vi "45-1523-1 State Diagram.vi"() -> ()   [LabVIEW 2015] (continued)
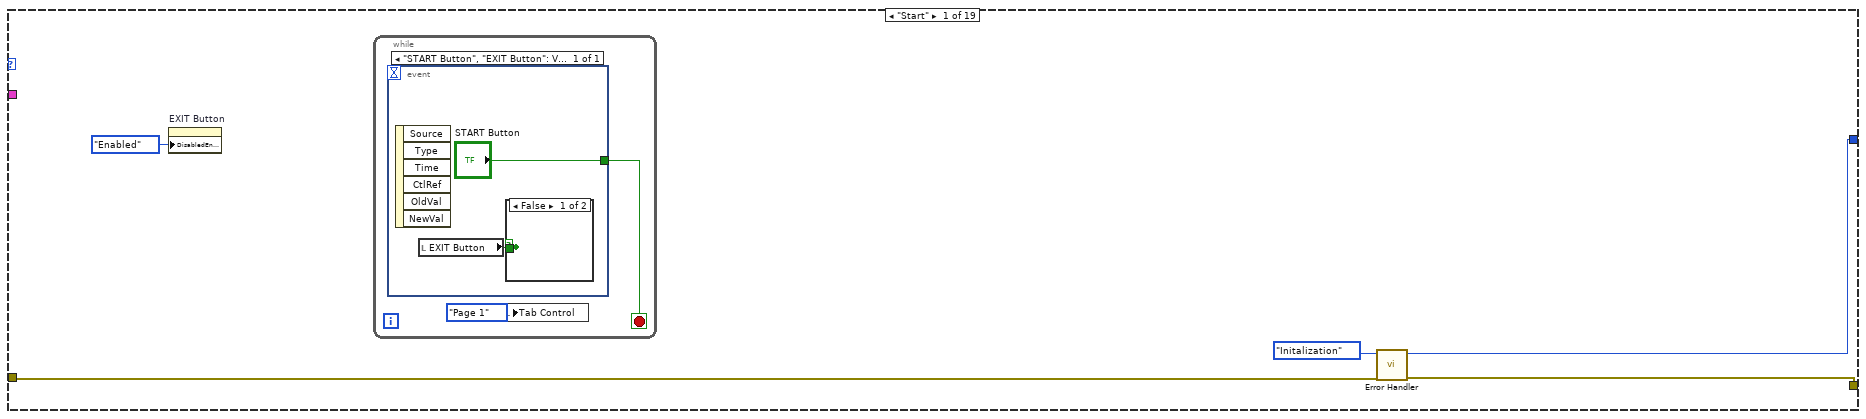
[diagram p2: hidden frame]
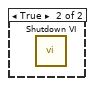
[diagram p3: hidden frame]
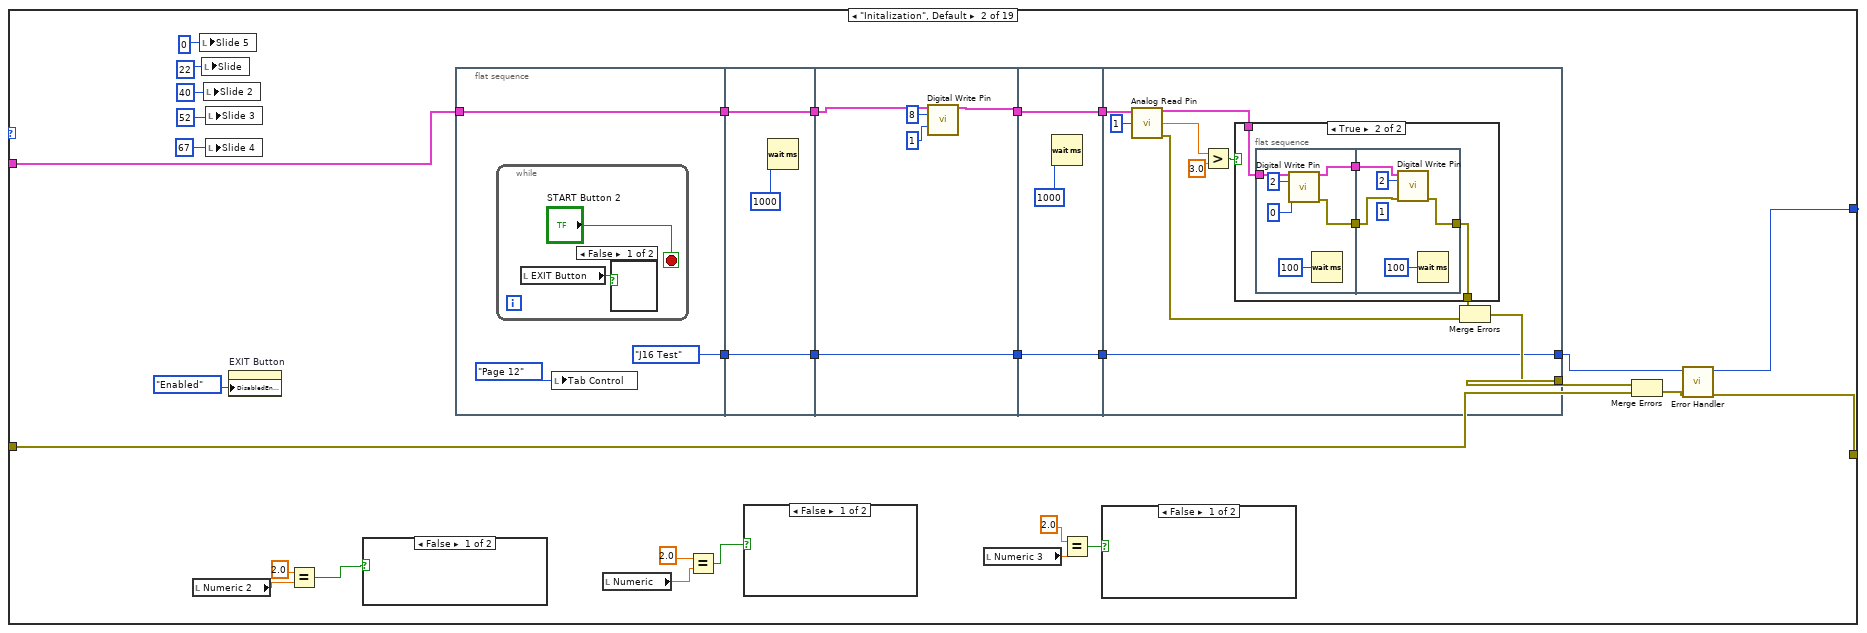
[diagram p4: hidden frame]
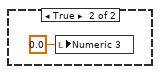
[diagram p5: hidden frame]
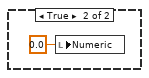
[diagram p6: hidden frame]
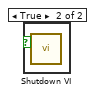
[diagram p7: hidden frame]
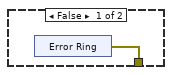
[diagram p8: hidden frame]
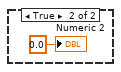
[diagram p9: hidden frame]
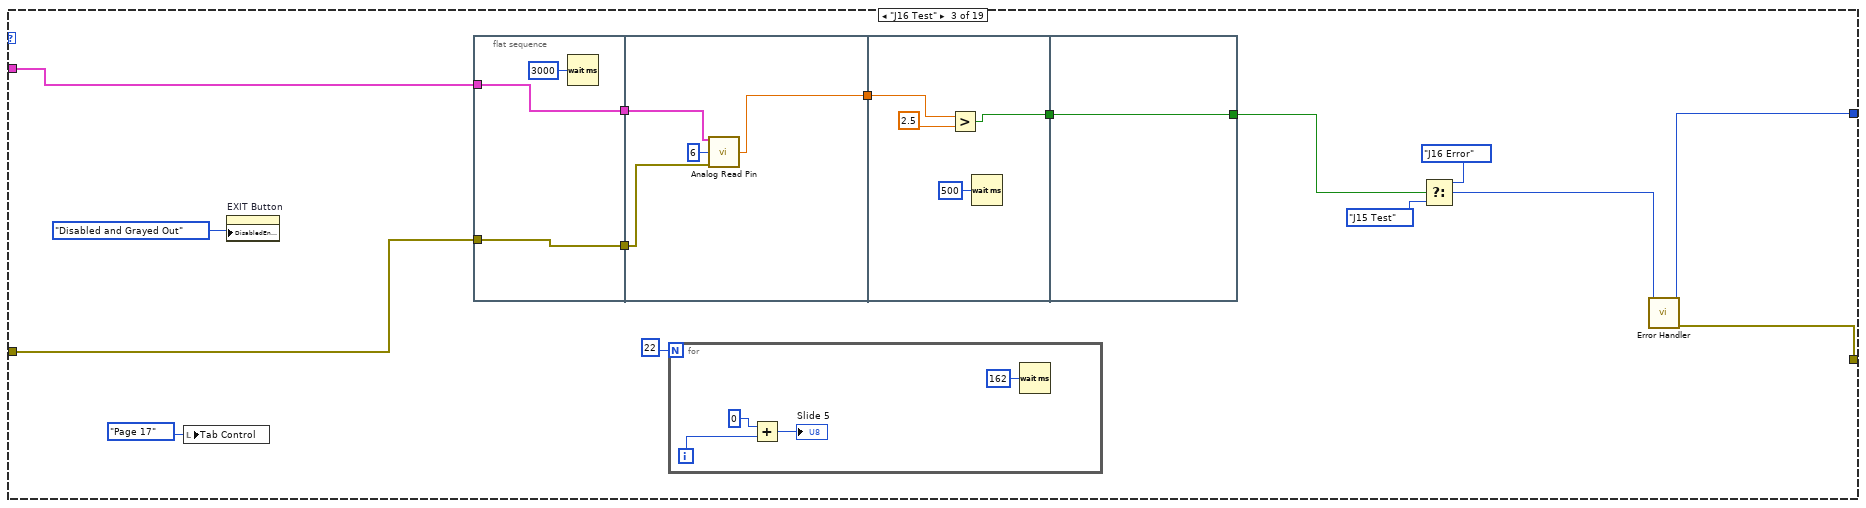
[diagram p10: hidden frame]
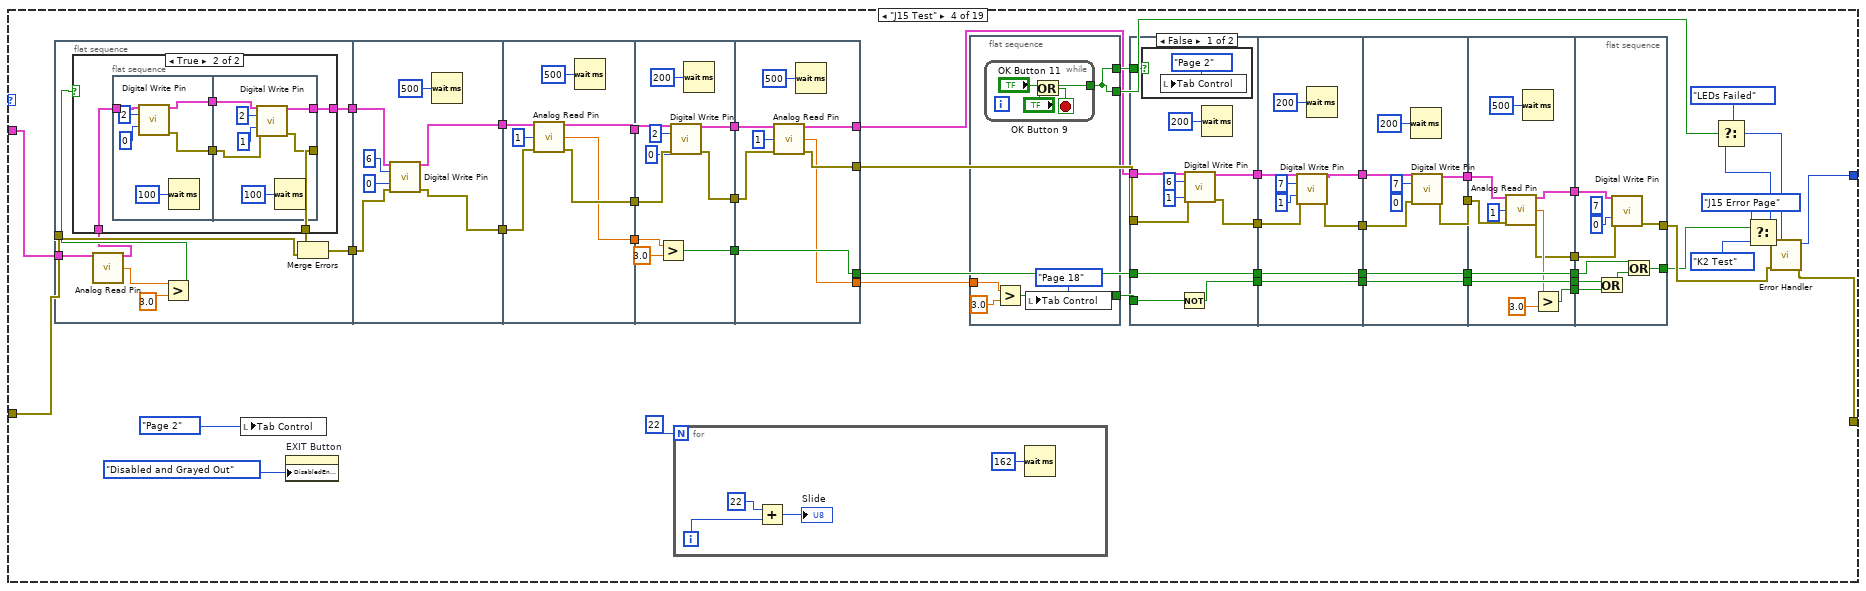
[diagram p11: hidden frame]
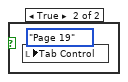
[diagram p12: hidden frame]
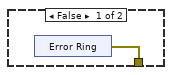
[diagram p13: hidden frame]
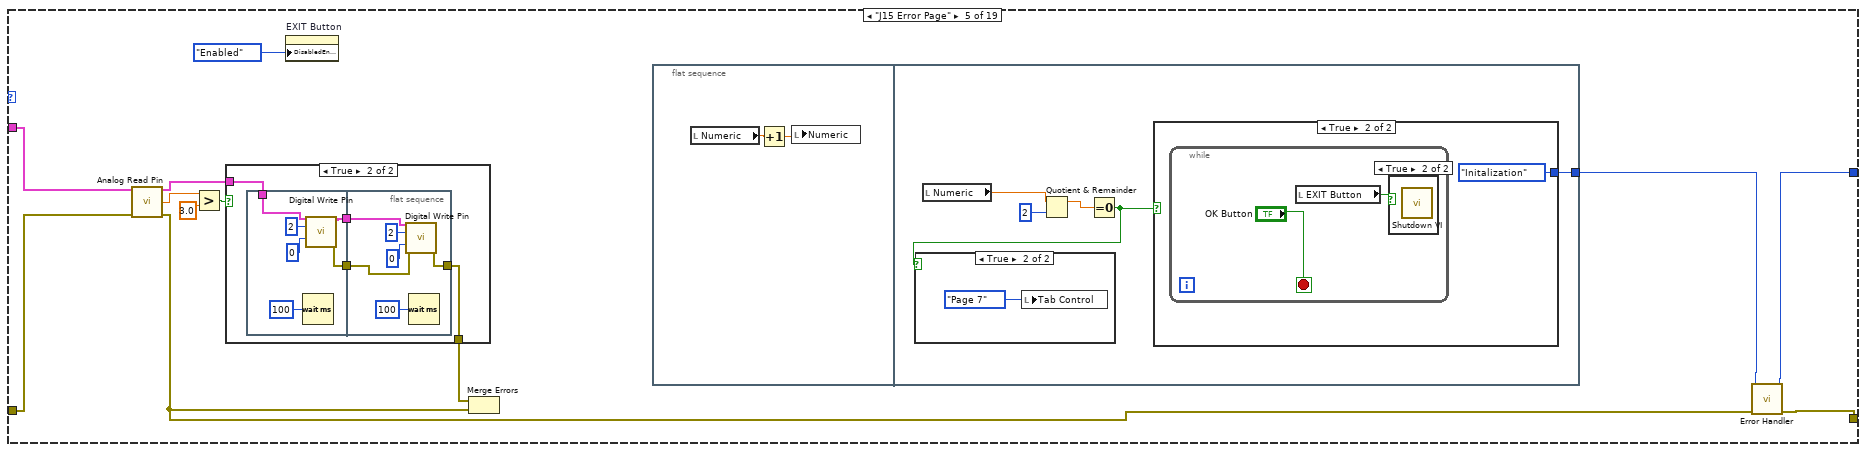
[diagram p14: hidden frame]
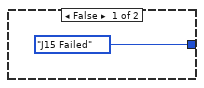
[diagram p16: hidden frame]
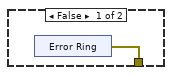
[diagram p18: hidden frame]
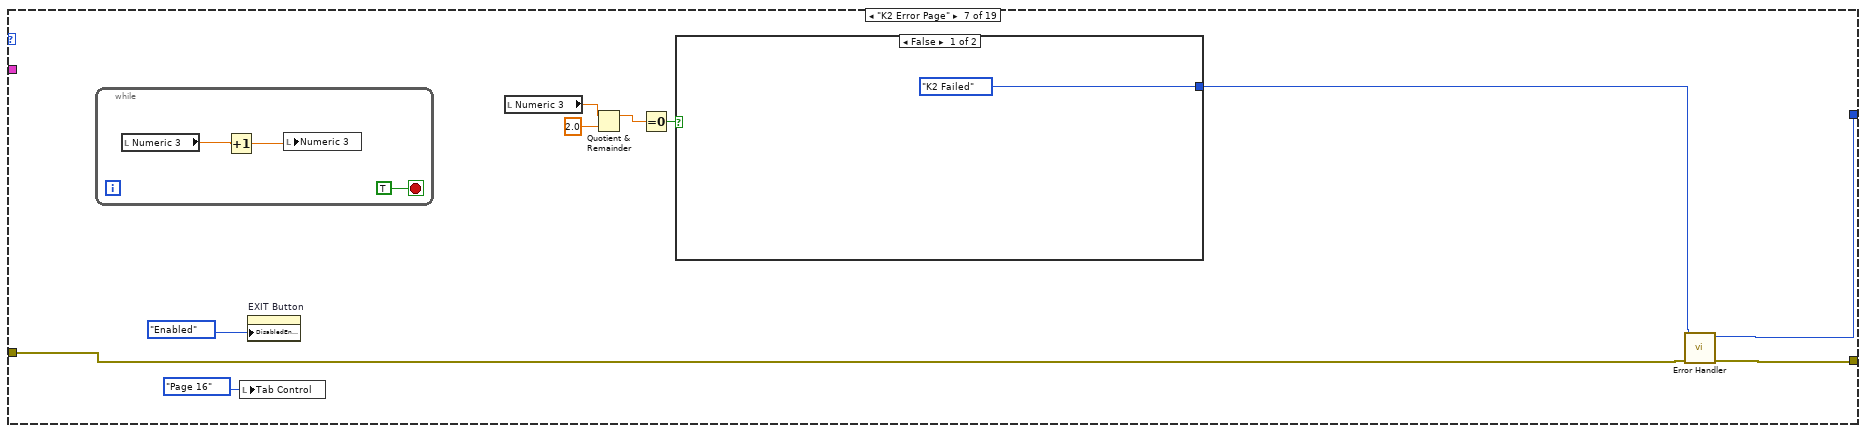
[diagram p19: hidden frame]
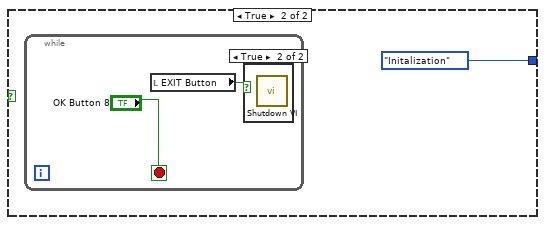
[diagram p20: hidden frame]
        n181 = Equal To 0?(x=w461) -> (x = 0?=w462:bool)
        n182 = case shown="False" w462 {
          tunnel: [Cases."K2 Failed" ("Enum") Cases."Initalization" ("Enum")] -> w459
          frame False {
          }
          frame True {
            n183 = while {
              stop <- "OK Button 8" stop-if-true
              n184 = local read "EXIT Button"() -> (w473:bool)
              n185 = case shown="True" w473 {
                frame False {
                }
                frame True {
                  n186 = call "Shutdown VI.vi"() -> ()  [unwired: 12 in]
                }
              }
            }
          }
        }
        n187 = call "Error Handler.vi"("error in (no error)"=w466, "Enum in"=w459) -> ("error out"=w465:errorcluster, "Enum out"=w464:T2)  [unwired: 8 in]
      }
      frame "K3 Test" {
        n188 = local write "Tab Control"(T6."Page 4" ("Tab Control")) -> ()
        n189 = flat-sequence {
          tunnel: w484 -> [w508]
          tunnel: [w507] -> w476
          tunnel: [w515] -> w501
          tunnel: [w511] -> w489
          tunnel: [w509] -> w488
          tunnel: w476 -> [w510]
          tunnel: [w521] -> w500
          tunnel: w501 -> [w521]
          tunnel: [w520] -> w499
          tunnel: w489 -> [w516]
          tunnel: w488 -> [w518]
          tunnel: [w517] -> w487
          tunnel: [w516] -> w477
          tunnel: w500 -> [w533]
          tunnel: [w531] -> w498
          tunnel: w499 -> [w531]
          tunnel: [w530] -> w497
          tunnel: [w528] -> w494
          tunnel: [w526] -> w490
          tunnel: w487 -> [w525]
          tunnel: [w524] -> w486
          tunnel: w477 -> [w526]
          tunnel: w498 -> [w541]
          tunnel: w497 -> [w540]
          tunnel: [w540] -> w496
          tunnel: w494 -> [w538]
          tunnel: [w534] -> w492
          tunnel: [w537] -> w491
          tunnel: w490 -> [w537]
          tunnel: w486 -> [w536]
          tunnel: [w535] -> w485
          tunnel: w496 -> [w552]
          tunnel: [w549] -> w493
          tunnel: w492 -> [w547]
          tunnel: w491 -> [w546]
          tunnel: w485 -> [w545]
          tunnel: [w544] -> w475
          frame #0 {
            n190 = call "Power Check.vi"() -> ("error out"=w506:errorcluster)  [unwired: 11 in]
            n191 = Merge Errors(w506, w508) -> (w507:errorcluster)
          }
          frame #1 {
            n192 = call-poly <vilib>:"DAQmx Read.vi"("task/channels in"=refnum<k21> "Is K3 Closed", "error in"=w510) -> ("task out"=w515:refnum<k21>, "data"=w512:dbl, "error out"=w509:errorcluster)  [unwired: 11 in]
            n193 = Greater?(x=w512, y=3.0) -> (0:w511:bool)
          }
          frame #2 {
            n194 = call-poly <vilib>:"DAQmx Write.vi"("task/channels in"=refnum<k21> "Fire K3" ("DAQmx Task Name"), "data"=FALSE, "error in"=w518) -> ("task out"=w520:refnum<k21>, "error out"=w517:errorcluster)  [unwired: 10 in, 1 out]
            n195 = Wait (ms)(milliseconds to wait=u32 800) -> ()  [unwired: 1 out]
          }
          frame #3 {
            n196 = call-poly <vilib>:"DAQmx Read.vi"("task/channels in"=w533, "error in"=w525) -> ("task out"=w530:refnum<k21>, "data"=w527:dbl, "error out"=w524:errorcluster)  [unwired: 11 in]
            n197 = Wait (ms)(milliseconds to wait=u32 1000) -> ()  [unwired: 1 out]
            n198 = Greater?(x=w527, y=3.0) -> (0:w528:bool)
          }
          frame #4 {
            n199 = Not(x=w538) -> (.not. x?=w534:bool)
            n200 = call-poly <vilib>:"DAQmx Write.vi"("task/channels in"=w541, "data"=TRUE, "error in"=w536) -> ("error out"=w535:errorcluster)  [unwired: 10 in, 2 out]
            n201 = Wait (ms)(milliseconds to wait=u32 500) -> ()  [unwired: 1 out]
          }
          frame #5 {
            n202 = call-poly <vilib>:"DAQmx Read.vi"("task/channels in"=w552, "error in"=w545) -> ("data"=w550:dbl, "error out"=w544:errorcluster)  [unwired: 11 in, 1 out]
            n203 = Greater?(x=w550, y=3.0) -> (0:w548:bool)
            n204 = Or(x=w547, y=w548) -> (x .or. y?=w543:bool)
            n205 = Or(x=w546, y=w543) -> (x .or. y?=w549:bool)
          }
        }
        n206 = for {
          N: 14 -> [_]
          i -> [w504]
          n207 = Add(x=56, y=w504) -> (x+y=→"Slide 3":i32)
          n208 = Wait (ms)(milliseconds to wait=u32 162) -> ()  [unwired: 1 out]
        }
        n209 = Select(t=Cases."K3 Error Page" ("Enum"), s=w493, f=Cases."K4 Test" ("Enum")) -> (s? t:f=w480:T2)
        n210 = call "Error Handler.vi"("error in (no error)"=w475, "Enum in"=w480) -> ("error out"=w481:errorcluster, "Enum out"=w479:T2)  [unwired: 8 in]
      }
      frame "K3 Error Page" {
        n211 = local write "Tab Control"(T6."Page 9" ("Tab Control")) -> ()
        n212 = property on="EXIT Button" class="Bool (strict)"("DisabledEnum"=T5."Enabled" ("Disabled")) -> ()  [unwired: 2 in, 2 out]
        n213 = while {
          stop <- "OK Button 3" stop-if-true
          n214 = local read "EXIT Button"() -> (w559:bool)
          n215 = case shown="False" w559 {
            frame False {
            }
            frame True {
              n216 = call "Shutdown VI.vi"() -> ()  [unwired: 12 in]
            }
          }
        }
        n217 = call "Error Handler.vi"("error in (no error)"=w555, "Enum in"=Cases."Test Failed" ("Enum")) -> ("error out"=w556:errorcluster, "Enum out"=w553:T2)  [unwired: 8 in]
      }
      frame "K4 Test" {
        n218 = local write "Tab Control"(T6."Page 5" ("Tab Control")) -> ()
        n219 = flat-sequence {
          tunnel: w580 -> [w591]
          tunnel: [w588] -> w569
          tunnel: [w593] -> w572
          tunnel: w569 -> [w594]
          tunnel: [w592] -> w563
          tunnel: [w601] -> w581
          tunnel: w572 -> [w597]
          tunnel: [w597] -> w571
          tunnel: [w598] -> w567
          tunnel: w563 -> [w600]
          tunnel: [w612] -> w583
          tunnel: w581 -> [w612]
          tunnel: w571 -> [w611]
          tunnel: w567 -> [w606]
          tunnel: [w609] -> w565
          tunnel: [w605] -> w562
          tunnel: [w604] -> w561
          tunnel: w583 -> [w621]
          tunnel: [w618] -> w579
          tunnel: [w616] -> w570
          tunnel: w565 -> [w615]
          tunnel: [w615] -> w564
          tunnel: w562 -> [w614]
          tunnel: w561 -> [w619]
          tunnel: w579 -> [w626]
          tunnel: w570 -> [w624]
          tunnel: [w625] -> w568
          tunnel: [w632] -> w566
          tunnel: w564 -> [w629]
          frame #0 {
            n220 = call "Power Check.vi"() -> ("error out"=w590:errorcluster)  [unwired: 11 in]
            n221 = Merge Errors(w590, w591) -> (w588:errorcluster)
            n222 = Wait (ms)(milliseconds to wait=u32 800) -> ()  [unwired: 1 out]
          }
          frame #1 {
            n223 = call "DAQ Assistant2"("error in"=w594) -> ("data"=w595:dynamicdata)  [unwired: 16 in, 2 out]
            n224 = call "Amplitude and Level Measurements"("Signals"=w595) -> ("Peak to Peak"=w596:dynamicdata, "error out"=w592:errorcluster)  [unwired: 1 in, 12 out]
            n225 = call "Convert from Dynamic Data4"("Dynamic Data Type"=w596) -> ("Scalar"=w593:dbl)  [unwired: 3 in]
          }
          frame #2 {
            n226 = call-poly <vilib>:"DAQmx Write.vi"("task/channels in"=refnum<k21> "Fire K4" ("DAQmx Task Name"), "data"=FALSE, "error in"=w600) -> ("task out"=w601:refnum<k21>, "error out"=w598:errorcluster)  [unwired: 10 in, 1 out]
            n227 = Wait (ms)(milliseconds to wait=u32 500) -> ()  [unwired: 1 out]
          }
          frame #3 {
            n228 = call "DAQ Assistant3"("error in"=w606) -> ("data"=w607:dynamicdata)  [unwired: 16 in, 2 out]
            n229 = Greater?(x=w611, y=0.08) -> (0:w609:bool)
            n230 = Wait (ms)(milliseconds to wait=u32 800) -> ()  [unwired: 1 out]
            n231 = call "Amplitude and Level Measurements2"("Signals"=w607) -> ("Peak to Peak"=w608:dynamicdata, "error out"=w604:errorcluster)  [unwired: 1 in, 12 out]
            n232 = call "Convert from Dynamic Data"("Dynamic Data Type"=w608) -> ("Scalar"=w605:dbl)  [unwired: 3 in]
          }
          frame #4 {
            n233 = Less?(x=w614, y=0.08) -> (x < y?=w616:bool)
            n234 = call-poly <vilib>:"DAQmx Write.vi"("task/channels in"=w621, "data"=TRUE, "error in"=w619) -> ("error out"=w618:errorcluster)  [unwired: 10 in, 2 out]
            n235 = Wait (ms)(milliseconds to wait=u32 500) -> ()  [unwired: 1 out]
          }
          frame #5 {
            n236 = call "DAQ Assistant4"("error in"=w626) -> ("data"=w627:dynamicdata)  [unwired: 16 in, 2 out]
            n237 = call "Amplitude and Level Measurements3"("Signals"=w627) -> ("Peak to Peak"=w628:dynamicdata, "error out"=w625:errorcluster)  [unwired: 1 in, 12 out]
            n238 = call "Convert from Dynamic Data2"("Dynamic Data Type"=w628) -> ("Scalar"=w623:dbl)  [unwired: 3 in]
            n239 = Greater?(x=w623, y=0.08) -> (0:w630:bool)
            n240 = Or(x=w624, y=w630) -> (x .or. y?=w633:bool)
            n241 = Or(x=w629, y=w633) -> (x .or. y?=w632:bool)
          }
        }
        n242 = for {
          N: 30 -> [_]
          i -> [w586]
          n243 = Add(x=70, y=w586) -> (x+y=→"Slide 4":i32)
          n244 = Wait (ms)(milliseconds to wait=u32 162) -> ()  [unwired: 1 out]
        }
        n245 = Select(t=Cases."K4 Error Page" ("Enum"), s=w566, f=Cases."Test Complete" ("Enum")) -> (s? t:f=w576:T2)
        n246 = call "Error Handler.vi"("error in (no error)"=w568, "Enum in"=w576) -> ("error out"=w574:errorcluster, "Enum out"=w575:T2)  [unwired: 8 in]
      }
      frame "K4 Error Page" {
        n247 = local write "Tab Control"(T6."Page 10" ("Tab Control")) -> ()
        n248 = property on="EXIT Button" class="Bool (strict)"("DisabledEnum"=T5."Enabled" ("Disabled")) -> ()  [unwired: 2 in, 2 out]
        n249 = while {
          stop <- "OK Button 4" stop-if-true
          n250 = local read "EXIT Button"() -> (w640:bool)
          n251 = case shown="True" w640 {
            frame False {
            }
            frame True {
              n252 = call "Shutdown VI.vi"() -> ()  [unwired: 12 in]
            }
          }
        }
        n253 = call "Error Handler.vi"("error in (no error)"=w634, "Enum in"=Cases."Test Failed" ("Enum")) -> ("error out"=w635:errorcluster, "Enum out"=w636:T2)  [unwired: 8 in]
      }
      frame "Test Complete" {
        n254 = local write "Tab Control"(T6."Page 6" ("Tab Control")) -> ()
        n255 = property on="EXIT Button" class="Bool (strict)"("DisabledEnum"=T5."Enabled" ("Disabled")) -> ()  [unwired: 2 in, 2 out]
        n256 = local write "Numeric 2"(0.0 ("Numeric 2")) -> ()
        n257 = event shown="[0] \"Restart Button\", \"EXIT Button\": Value Change" {
          selector: _ -> [_]
          dyn-events: _ -> [_]
          timeout: _ -> [_]
          tunnel: [Cases."Start" ("Enum")] -> w646
          event "Restart Button", "EXIT Button": Value Change {
            n258 = event-data() -> ()  [unwired: 1 in, 6 out]
            n259 = while {
              stop <- "Restart Button" stop-if-true
              n260 = local read "EXIT Button"() -> (w650:bool)
              n261 = case shown="True" w650 {
                frame False {
                }
                frame True {
                  n262 = call "Shutdown VI.vi"() -> ()  [unwired: 12 in]
                }
              }
            }
          }
        }
        n263 = call "Error Handler.vi"("error in (no error)"=w643, "Enum in"=w646) -> ("error out"=w644:errorcluster, "Enum out"=w645:T2)  [unwired: 8 in]
      }
      frame "Test Failed" {
        n264 = local write "Tab Control"(T6."Page 11" ("Tab Control")) -> ()
        n265 = call-poly <vilib>:"DAQmx Read.vi"("task/channels in"=refnum<k21> "Is J15 Closed") -> ("data"=w658:dbl, "error out"=w654:errorcluster)  [unwired: 12 in, 1 out]
        n266 = Greater?(x=w658, y=3.0) -> (0:w656:bool)
        n267 = case shown="True" w656 {
          tunnel: [w664 w666] -> w655
          frame False {
            n268 = xnode "Error Ring"() -> ("error out"=w664:errorcluster)
          }
          frame True {
            n269 = flat-sequence {
              tunnel: [w670] -> w667
              tunnel: [w675] -> w666
              tunnel: w667 -> [w676]
              frame #0 {
                n270 = call-poly <vilib>:"DAQmx Write.vi"("task/channels in"=refnum<k21> "Fire K1", "data"=FALSE) -> ("error out"=w670:errorcluster)  [unwired: 11 in, 2 out]
                n271 = Wait (ms)(milliseconds to wait=u32 100) -> ()  [unwired: 1 out]
              }
              frame #1 {
                n272 = call-poly <vilib>:"DAQmx Write.vi"("task/channels in"=refnum<k21> "Fire K1", "data"=TRUE, "error in"=w676) -> ("error out"=w675:errorcluster)  [unwired: 10 in, 2 out]
                n273 = Wait (ms)(milliseconds to wait=u32 100) -> ()  [unwired: 1 out]
              }
            }
          }
        }
        n274 = Merge Errors(w655, w654, w653) -> (w652:errorcluster)
        n275 = event shown="[0] \"EXIT Button\", \"Restart Button 2\": Value Change" {
          selector: _ -> [_]
          dyn-events: _ -> [_]
          timeout: _ -> [_]
          event "EXIT Button", "Restart Button 2": Value Change {
            n276 = event-data() -> ()  [unwired: 1 in, 6 out]
            n277 = while {
              stop <- "Restart Button 2" stop-if-true
              n278 = local read "EXIT Button"() -> (w677:bool)
              n279 = case shown="False" w677 {
                frame False {
                }
                frame True {
                  n280 = call "Shutdown VI.vi"() -> ()  [unwired: 12 in]
                }
              }
            }
          }
        }
        n281 = call "Error Handler.vi"("error in (no error)"=w652, "Enum in"=Cases."Start" ("Enum")) -> ("error out"=w660:errorcluster, "Enum out"=w661:T2)  [unwired: 8 in]
      }
      frame "Error" {
        n282 = case shown="No Error" w679 {
          tunnel: [w684 w689] -> w681
          tunnel: [w682 w687] -> w680
          tunnel: w679 -> [w685 w686]
          frame No Error {
            n283 = call "Error Handler.vi"("error in (no error)"=w685, "Enum in"=Cases."Initalization") -> ("error out"=w684:errorcluster, "Enum out"=w682:T2)  [unwired: 8 in]
          }
          frame Error {
            n284 = call <vilib>:"Clear Errors.vi"("error in (no error)"=w686, "specific error code to clear (0: all)"=0) -> ("error out"=w690:errorcluster)  [unwired: 4 in, 1 out]
            n285 = call "Error Handler.vi"("error in (no error)"=w690, "Enum in"=Cases."Error" ("Enum")) -> ("error out"=w689:errorcluster, "Enum out"=w687:T2)  [unwired: 8 in]
          }
        }
      }
      frame "J15 Failed" {
        n286 = local write "Tab Control"(T11."Page 13" ("Tab Control")) -> ()
        n287 = property on="EXIT Button" class="Bool (strict)"("DisabledEnum"=T5."Enabled" ("Disabled")) -> ()  [unwired: 2 in, 2 out]
        n288 = while {
          stop <- "OK Button 5" stop-if-true
          n289 = local read "EXIT Button"() -> (w698:bool)
          n290 = case shown="True" w698 {
            frame False {
            }
            frame True {
              n291 = call "Shutdown VI.vi"() -> ()  [unwired: 12 in]
            }
          }
        }
        n292 = call "Error Handler.vi"("error in (no error)"=w692, "Enum in"=Cases."Test Failed" ("Enum")) -> ("error out"=w693:errorcluster, "Enum out"=w694:T2)  [unwired: 8 in]
      }
      frame "J16 Error" {
        n293 = while {
          stop <- TRUE stop-if-true
          n294 = local read "Numeric 2"() -> (w715:dbl)
          n295 = Increment(x=w715) -> (x+1=w714:dbl)
          n296 = local write "Numeric 2"(w714) -> ()
        }
        n297 = local write "Tab Control"(T12."Page 14" ("Tab Control")) -> ()
        n298 = property on="EXIT Button" class="Bool (strict)"("DisabledEnum"=T5."Enabled" ("Disabled")) -> ()  [unwired: 2 in, 2 out]
        n299 = local read "Numeric 2"() -> (w702:dbl)
        n300 = Quotient & Remainder(x=w702, y=2.0) -> (x-y*floor(x/y)=w703:dbl)  [unwired: 1 out]
        n301 = Equal To 0?(x=w703) -> (x = 0?=w704:bool)
        n302 = case shown="True" w704 {
          tunnel: [Cases."J16 Failed" ("Enum") Cases."Initalization" ("Enum")] -> w700
          frame False {
          }
          frame True {
            n303 = while {
              stop <- "OK Button 6" stop-if-true
              n304 = local read "EXIT Button"() -> (w712:bool)
              n305 = case shown="False" w712 {
                frame False {
                }
                frame True {
                  n306 = call "Shutdown VI.vi"() -> ()  [unwired: 12 in]
                }
              }
            }
          }
        }
        n307 = call "Error Handler.vi"("error in (no error)"=w707, "Enum in"=w700) -> ("error out"=w708:errorcluster, "Enum out"=w706:T2)  [unwired: 8 in]
      }
      frame "J16 Failed" {
        n308 = local write "Tab Control"(T13."Page 15" ("Tab Control")) -> ()
        n309 = property on="EXIT Button" class="Bool (strict)"("DisabledEnum"=T5."Enabled" ("Disabled")) -> ()  [unwired: 2 in, 2 out]
        n310 = while {
          stop <- "OK Button 7" stop-if-true
          n311 = local read "EXIT Button"() -> (w723:bool)
          n312 = case shown="True" w723 {
            frame False {
            }
            frame True {
              n313 = call "Shutdown VI.vi"() -> ()  [unwired: 12 in]
            }
          }
        }
        n314 = call "Error Handler.vi"("error in (no error)"=w720, "Enum in"=Cases."Test Failed" ("Enum")) -> ("error out"=w719:errorcluster, "Enum out"=w717:T2)  [unwired: 8 in]
      }
      frame "K2 Failed" {
        n315 = local write "Tab Control"(T10."Page 8" ("Tab Control")) -> ()
        n316 = property on="EXIT Button" class="Bool (strict)"("DisabledEnum"=T5."Enabled" ("Disabled")) -> ()  [unwired: 2 in, 2 out]
        n317 = while {
          stop <- "OK Button 10" stop-if-true
          n318 = local read "EXIT Button"() -> (w732:bool)
          n319 = case shown="True" w732 {
            frame False {
            }
            frame True {
              n320 = call "Shutdown VI.vi"() -> ()  [unwired: 12 in]
            }
          }
        }
        n321 = call "Error Handler.vi"("error in (no error)"=w726, "Enum in"=Cases."Test Failed") -> ("error out"=w725:errorcluster, "Enum out"=w727:T2)  [unwired: 8 in]
      }
      frame "LEDs Failed" {
        n322 = local write "Tab Control"(T1."Page 19" ("Tab Control")) -> ()
        n323 = property on="EXIT Button" class="Bool (strict)"("DisabledEnum"=T5."Enabled" ("Disabled")) -> ()  [unwired: 2 in, 2 out]
        n324 = while {
          stop <- "OK Button 12" stop-if-true
          n325 = local read "EXIT Button"() -> (w739:bool)
          n326 = case shown="True" w739 {
            frame False {
            }
            frame True {
              n327 = call "Shutdown VI.vi"() -> ()  [unwired: 12 in]
            }
          }
        }
        n328 = call "Error Handler.vi"("error in (no error)"=w736, "Enum in"=Cases."Test Failed") -> ("error out"=w737:errorcluster, "Enum out"=w735:T2)  [unwired: 8 in]
      }
    }
  }
